vi "string parse mathematica list assosiated array.vi"(6 "pattern":string="[\\\\\\s\\n]*(\\d+)[\\\\\\s\\n]*\\-\\>[\\\\\\s\\n]*\\<\\|((.|\\n)+?)\\|\\>[\\\\\\s\\n]*\\,", 7 "derivative":T2=enum."parse string", 8 "array of inds":dbl[](array[numeric]), 10 "Map IN":map{i32, map{T1, dbl}}(c390), 11 "string IN":string) -> (2 "Map OUT":map{i32, map{T1, dbl}}(c390), 3 "string out":string)   [LabVIEW 2020]
uses:
  3-lorentzian-parameters.ctl
  3-lorentzian-heat-response action.ctl
  mathematica string map action.ctl
  3-lorentzian-heat-response -- V4.vi/142dd4c5-f9ed-c64b-bc14-a88e3e2c450a.vi
  <vilib>/Analysis/polynomials.llb/Multiply Polynomials.vi
  <vilib>/Analysis/polynomials.llb/Multiply Polynomials (DBL).vi
  <vilib>/Analysis/polynomials.llb/Polynomial Roots.vi
  <vilib>/Analysis/polynomials.llb/Polynomial Roots (DBL).vi
  <vilib>/Comparison/Less/Less Functor/Less Functor.lvclass
  <vilib>/regexp/Match Regular Expression.xnode
panel:
  out "after match":string
  out "map of strings":map{i32, string}(c390)
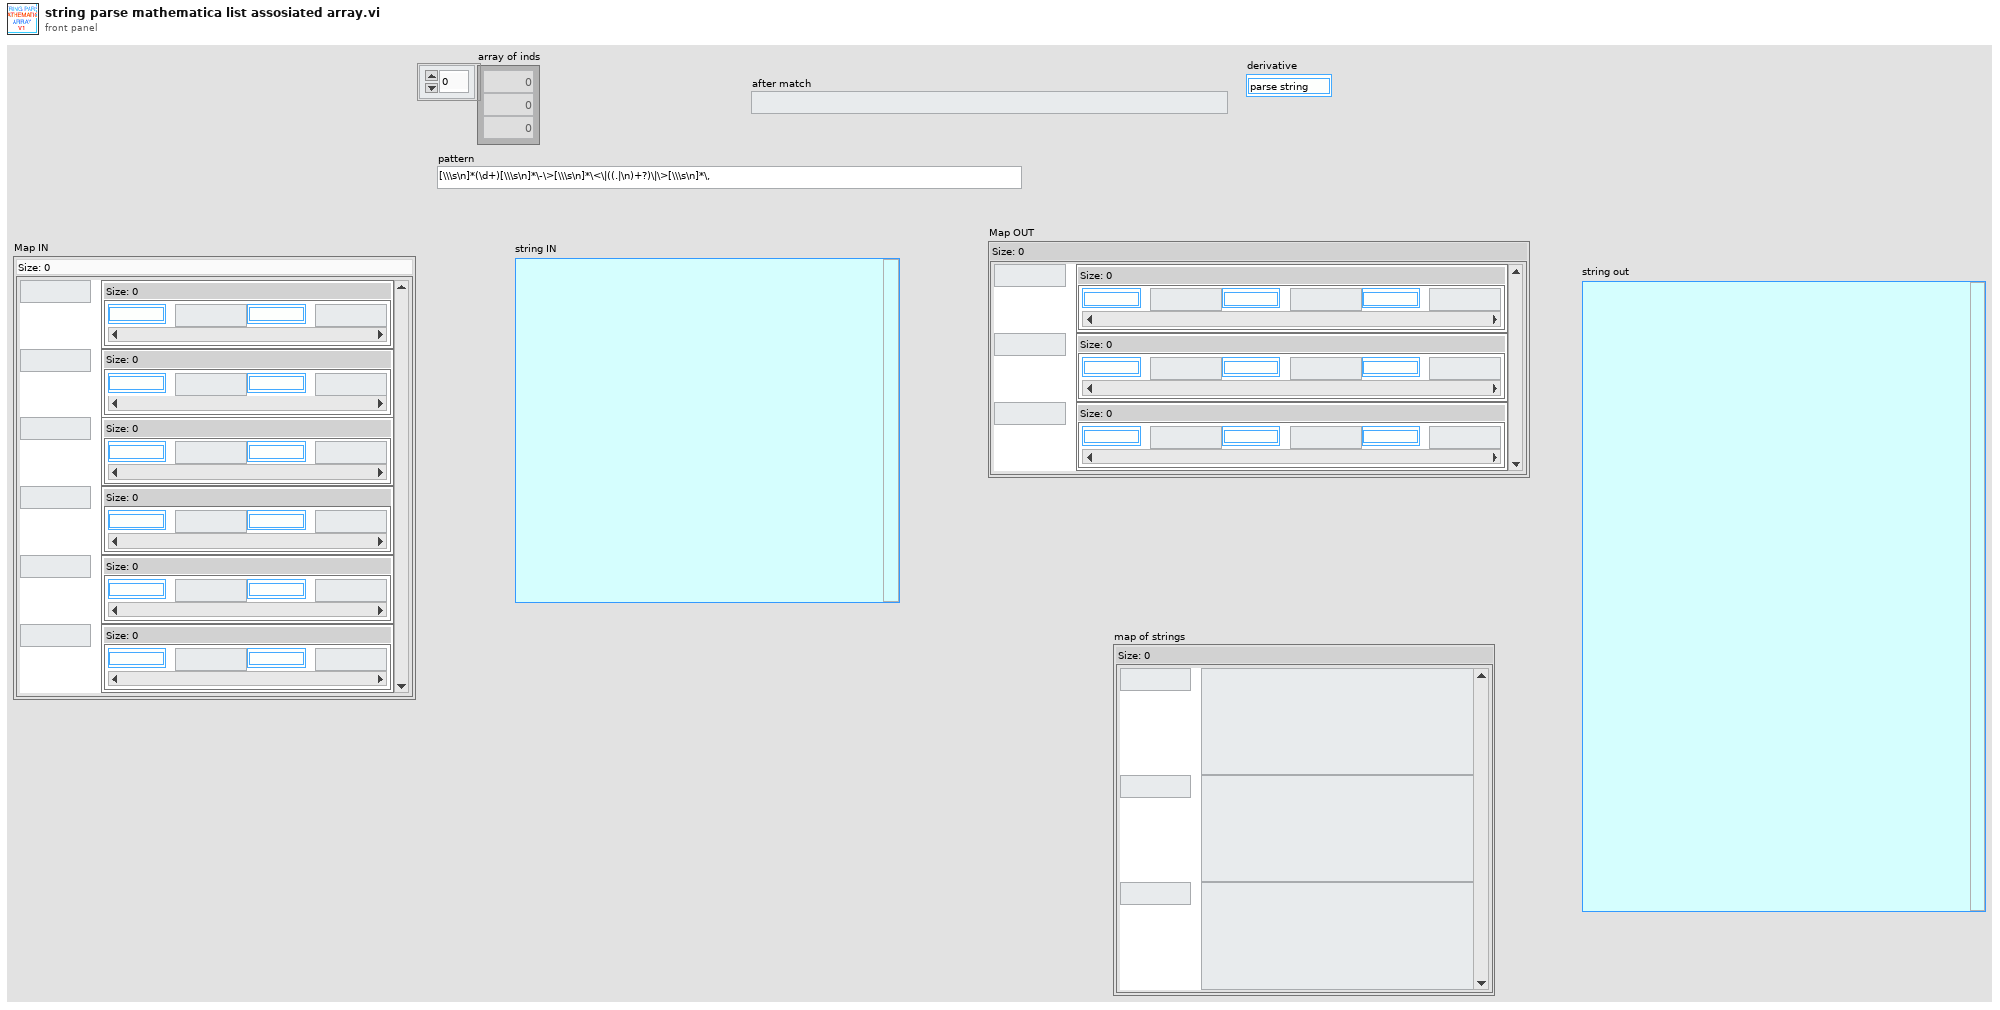
[diagram p1: front panel]
types:
  T1 = typedef "3-lorentzian-parameters.ctl" = enum16{"ζ", "τ1", "τS", "τN", "τC", "κ0", "m1", "m2", "m3", "T (K)", "B (T)", "θ (deg)", "side (S|R)", "set of (B|T)", "Re(offset)", "Im(offset)"}
  T2 = typedef "3-lorentzian-heat-response action.ctl" = enum16{"calc R", "create string", "calc m1m2m3", "dζ", "dT1", "dτS", "dτN", "dτC", "d-all", "dκ0", "T(K)", "m1", "m2", "m3", "parse string", "θ (deg)", "B (T)", "onlygrads", "newton", "create emty string"}
  T3 = typedef "mathematica string map action.ctl" = enum16{"create string", "calc m1m2m3", "parse string"}
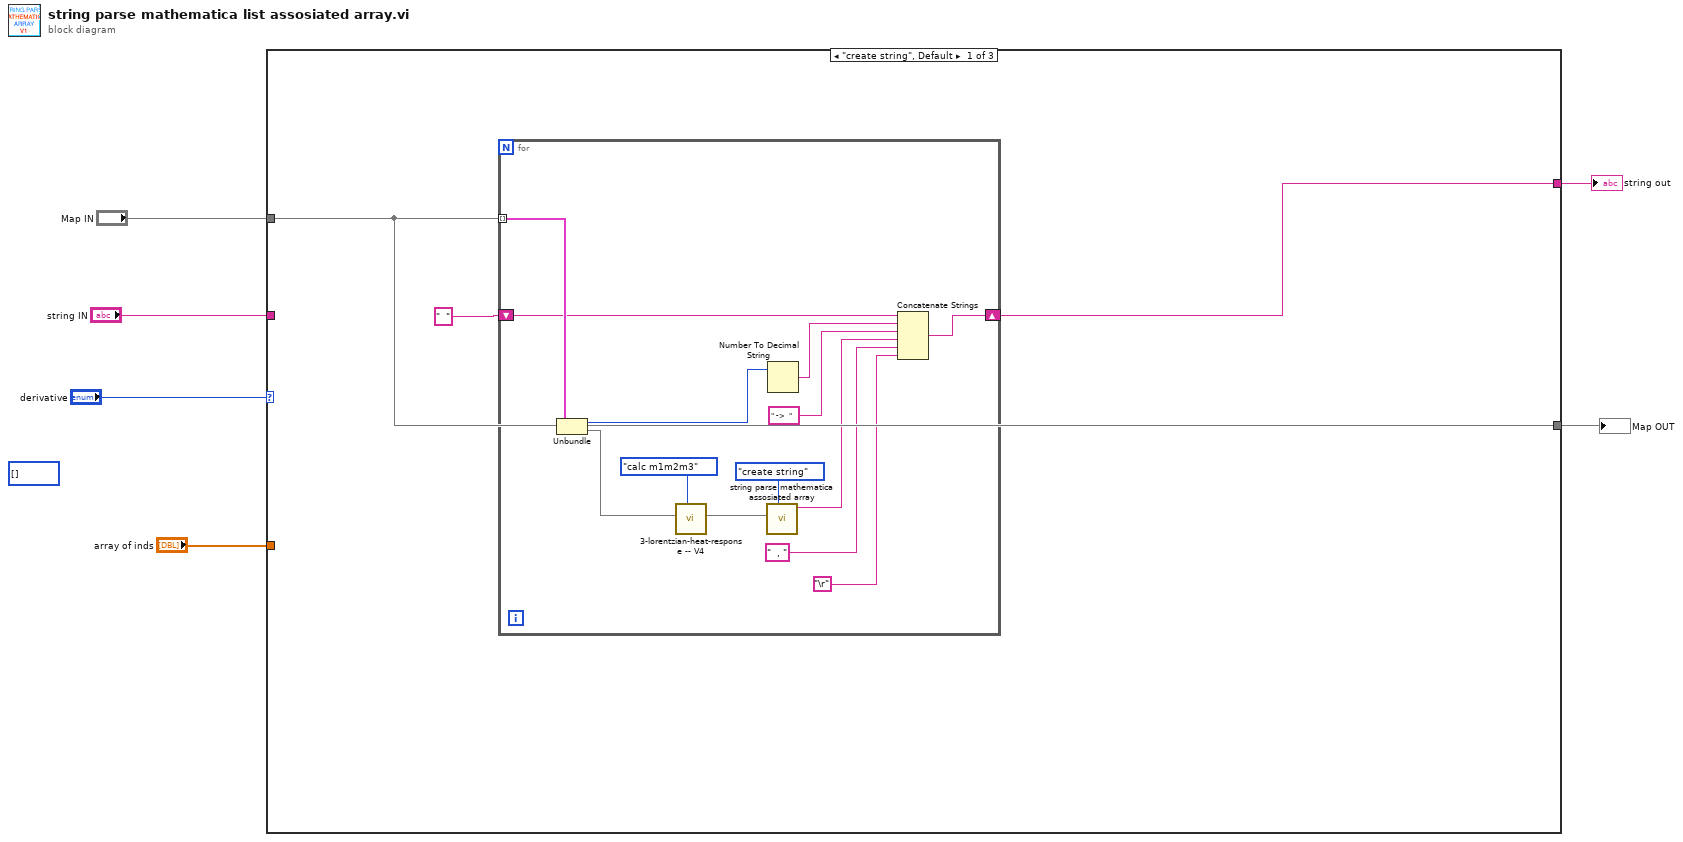
[diagram p0: block diagram]
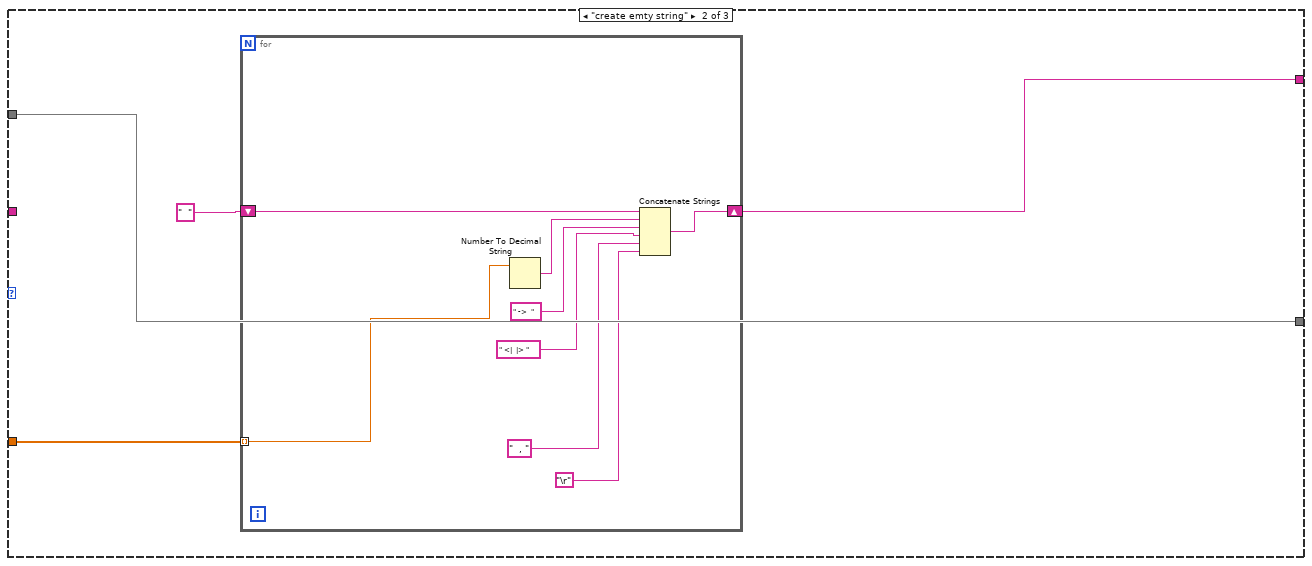
[diagram p2: hidden frame]
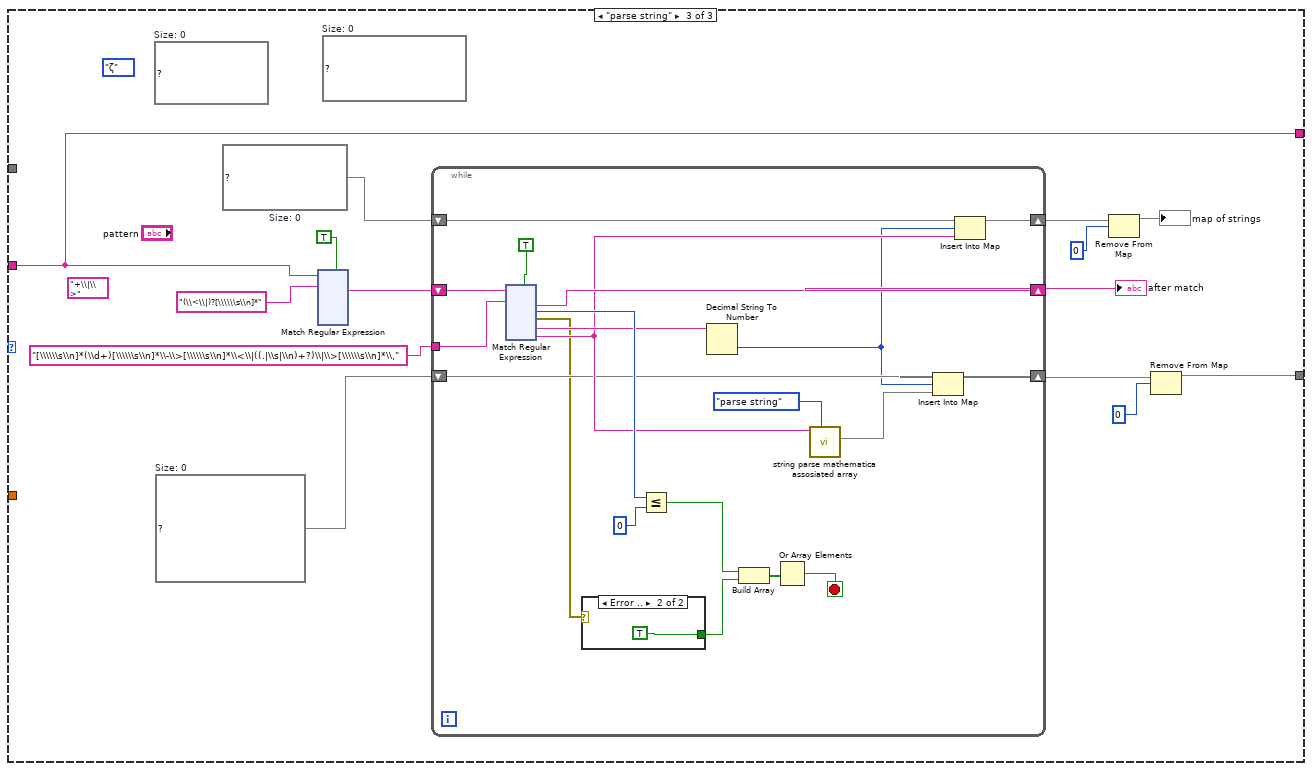
[diagram p3: hidden frame]
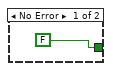
[diagram p4: hidden frame]
diagram:
  (unwired) i32[] []
  n1 = case shown="\"create string\", Default" "derivative" {
    tunnel: "string IN" -> [_ _ w37]
    tunnel: [w7 w24 w38] -> w5
    tunnel: "Map IN" -> [w7 w24 _]
    tunnel: [w9 w26 w37] -> w2
    tunnel: "array of inds" -> [_ w23 _]
    frame "create string", Default {
      n2 = for {
        tunnel: w7 -> [w22] mode=indexing
        shift-right: [w14] -> w9
        shift-left: "  " ("all string") -> [w15]
        n3 = Unbundle(w22) -> ("index"=w21:i32, "Map"=w12:map{T1, dbl})
        n4 = call "3-lorentzian-heat-response -- V4.vi"("action"=3-lorentzian-heat-response_action."calc m1m2m3", "Map IN"=w12) -> ("Map OUT"=w10:map{T1, dbl})  [unwired: 7 in, 2 out]
        n5 = call "string parse mathematica assosiated array.vi"("action"=mathematica_string_map_action."create string" ("derivative"), "map IN"=w10) -> ("String OUT"=w18:string)  [unwired: 8 in, 1 out]
        n6 = Number To Decimal String(number=w21) -> (decimal integer string=w20:string)  [unwired: 1 in]
        n7 = Concatenate Strings(w15, w20, " ->  " ("all string"), w18, "  , " ("all string"), "\r") -> (w14:string)
      }
    }
    frame "create emty string" {
      n8 = for {
        shift-right: [w30] -> w26
        shift-left: "  " ("all string") -> [w31]
        tunnel: w23 -> [w28] mode=indexing
        n9 = Number To Decimal String(number=w28) -> (decimal integer string=w34:string)  [unwired: 1 in]
        n10 = Concatenate Strings(w31, w34, " ->  " ("all string"), " <|  |> " ("all string"), "  , " ("all string"), "\r") -> (w30:string)
      }
    }
    frame "parse string" {
      (unwired) 3-lorentzian-parameters."ζ" ("X selector")
      w44 = map{i32, map{T1, dbl}} {}  # Size: 0
      w46 = map{i32, string} {}  # Size: 0
      (unwired) "+\\|\\>" ("format string")
      (unwired) map{T1, dbl} {}  # Size: 0
      (unwired) map{T1, string} {}  # Size: 0
      n11 = xnode "Match Regular Expression"("input string"=w37, "regular expression"="(\\<\\|)?[\\\\\\s\\n]*" ("format string"), "multiline? (F)"=TRUE) -> ("after match"=w47:string)  [unwired: 3 in, 6 out]
      n12 = while {
        shift-right: [w65] -> w45
        shift-left: w47 -> [w68]
        tunnel: "[\\\\\\s\\n]*(\\d+)[\\\\\\s\\n]*\\-\\>[\\\\\\s\\n]*\\<\\|((.|\\s|\\n)+?)\\|\\>[\\\\\\s\\n]*\\," ("pattern") -> [w64]
        shift-right: [w61] -> w43
        shift-left: w46 -> [w63]
        shift-right: [w55] -> w39
        shift-left: w44 -> [w58]
        stop <- w51 stop-if-true
        n13 = xnode "Match Regular Expression"("input string"=w68, "regular expression"=w64, "multiline? (F)"=TRUE) -> ("after match"=w65:string, "offset past match"=w67:i32, "error out"=w52:errorcluster, "submatch 1"=w62:string, "submatch 2"=w59:string)  [unwired: 3 in, 2 out]
        n14 = case shown="Error .." w52 {
          tunnel: [FALSE TRUE] -> w49
          frame No Error {
          }
          frame Error {
          }
        }
        n15 = Less Or Equal?(x=w67, y=0) -> (x <= y?=w53:bool)
        n16 = Decimal String To Number(string=w62) -> (number=w57:i32)  [unwired: 2 in, 1 out]
        n17 = Build Array(w53, w49) -> (w50:bool[])
        n18 = Or Array Elements(Boolean array=w50) -> (logical OR=w51:bool)
        n19 = call "string parse mathematica assosiated array.vi"("action"=mathematica_string_map_action."parse string" ("derivative"), "String in"=w59) -> ("Map OUT"=w56:map{T1, dbl})  [unwired: 8 in, 1 out]
        n20 = Insert Into Map(map in=w58, key=w57, value=w56) -> (map out=w55:map{i32, map{T1, dbl}})  [unwired: 2 out]
        n21 = Insert Into Map(map in=w63, key=w57, value=w59) -> (map out=w61:map{i32, string})  [unwired: 2 out]
      }
      "after match" <- w45
      n22 = Remove From Map(10:0 ("key"), 11:w43) -> (3:→"map of strings":map{i32, string})  [unwired: 2 out]
      n23 = Remove From Map(10:0 ("key"), 11:w39) -> (3:w38:map{i32, map{T1, dbl}})  [unwired: 2 out]
    }
  }
  "Map OUT" <- w5
  "string out" <- w2
